vi "HFRR ADV v040.vi"() -> ()   [LabVIEW 2025] (continued)
            n2198 = Delete From Array(array=w2502, index=0) -> (array with subset deleted=w2408:dbl[])  [unwired: 1 in, 1 out]
            n2199 = Delete From Array(array=w2448, index=0) -> (array with subset deleted=w2404:dbl[])  [unwired: 1 in, 1 out]
            n2200 = Delete From Array(array=w2484, index=0) -> (array with subset deleted=w2406:dbl[])  [unwired: 1 in, 1 out]
            n2201 = Delete From Array(array=w2444, index=0) -> (array with subset deleted=w2402:dbl[])  [unwired: 1 in, 1 out]
            n2202 = Delete From Array(array=w2493, index=0) -> (array with subset deleted=w2407:dbl[])  [unwired: 1 in, 1 out]
            n2203 = Delete From Array(array=w2446, index=0) -> (array with subset deleted=w2403:dbl[])  [unwired: 1 in, 1 out]
            n2204 = Delete From Array(array=w2427, index=0) -> (array with subset deleted=w2399:dbl[])  [unwired: 1 in, 1 out]
            n2205 = Delete From Array(array=w2471, index=0) -> (array with subset deleted=w2457:dbl[])  [unwired: 1 in, 1 out]
            n2206 = Delete From Array(array=w2498, index=0) -> (array with subset deleted=w2459:dbl[])  [unwired: 1 in, 1 out]
            n2207 = Delete From Array(array=w2475, index=0) -> (array with subset deleted=w2405:dbl[])  [unwired: 1 in, 1 out]
            n2208 = Delete From Array(array=w2442, index=0) -> (array with subset deleted=w2401:dbl[])  [unwired: 1 in, 1 out]
            n2209 = Delete From Array(array=w2423, index=0) -> (array with subset deleted=w2397:dbl[])  [unwired: 1 in, 1 out]
            n2210 = Delete From Array(array=w2467, index=0) -> (array with subset deleted=w2455:dbl[])  [unwired: 1 in, 1 out]
            n2211 = Delete From Array(array=w2480, index=0) -> (array with subset deleted=w2460:dbl[])  [unwired: 1 in, 1 out]
            n2212 = Delete From Array(array=w2490, index=0) -> (array with subset deleted=w2373:dbl[])  [unwired: 1 in, 1 out]
            n2213 = Delete From Array(array=w2500, index=0) -> (array with subset deleted=w2375:dbl[])  [unwired: 1 in, 1 out]
            n2214 = Delete From Array(array=w2482, index=0) -> (array with subset deleted=w2371:dbl[])  [unwired: 1 in, 1 out]
            n2215 = Bundle "Bundle"(w2377, w2408) -> (w2395:cluster{dbl[], dbl[]})  [unwired: 1 in]
            n2216 = Bundle "Bundle"(w2377, w2462) -> (w2396:cluster{dbl[], dbl[]})  [unwired: 1 in]
            n2217 = Bundle "Bundle"(w2408, w2404) -> (w2410:cluster{dbl[], dbl[]})  [unwired: 1 in]
            n2218 = Bundle "Bundle"(w2373, w2372) -> (w2380:cluster{dbl[], dbl[]})  [unwired: 1 in]
            n2219 = Bundle "Bundle"(w2406, w2402) -> (w2412:cluster{dbl[], dbl[]})  [unwired: 1 in]
            n2220 = Bundle "Bundle"(w2373, w2406) -> (w2516:cluster{dbl[], dbl[]})  [unwired: 1 in]
            n2221 = Bundle "Bundle"(w2373, w2402) -> (w2440:cluster{dbl[], dbl[]})  [unwired: 1 in]
            n2222 = Bundle "Bundle"(w2373, w2461) -> (w2526:cluster{dbl[], dbl[]})  [unwired: 1 in]
            n2223 = Bundle "Bundle"(w2373, w2456) -> (w2464:cluster{dbl[], dbl[]})  [unwired: 1 in]
            n2224 = Bundle "Bundle"(w2373, w2487) -> (w2511:cluster{dbl[], dbl[]})  [unwired: 1 in]
            n2225 = Bundle "Bundle"(w2407, w2403) -> (w2411:cluster{dbl[], dbl[]})  [unwired: 1 in]
            n2226 = Bundle "Bundle"(w2375, w2374) -> (w2381:cluster{dbl[], dbl[]})  [unwired: 1 in]
            n2227 = Bundle "Bundle"(w2375, w2407) -> (w2518:cluster{dbl[], dbl[]})  [unwired: 1 in]
            n2228 = Bundle "Bundle"(w2375, w2403) -> (w2441:cluster{dbl[], dbl[]})  [unwired: 1 in]
            n2229 = Bundle "Bundle"(w2375, w2457) -> (w2465:cluster{dbl[], dbl[]})  [unwired: 1 in]
            n2230 = Bundle "Bundle"(w2375, w2459) -> (w2527:cluster{dbl[], dbl[]})  [unwired: 1 in]
            n2231 = Bundle "Bundle"(w2375, w2496) -> (w2509:cluster{dbl[], dbl[]})  [unwired: 1 in]
            n2232 = Bundle "Bundle"(w2405, w2401) -> (w2413:cluster{dbl[], dbl[]})  [unwired: 1 in]
            n2233 = Bundle "Bundle"(w2371, w2370) -> (w2379:cluster{dbl[], dbl[]})  [unwired: 1 in]
            n2234 = Bundle "Bundle"(w2371, w2405) -> (w2517:cluster{dbl[], dbl[]})  [unwired: 1 in]
            n2235 = Bundle "Bundle"(w2371, w2401) -> (w2439:cluster{dbl[], dbl[]})  [unwired: 1 in]
            n2236 = Bundle "Bundle"(w2371, w2455) -> (w2463:cluster{dbl[], dbl[]})  [unwired: 1 in]
            n2237 = Bundle "Bundle"(w2371, w2460) -> (w2525:cluster{dbl[], dbl[]})  [unwired: 1 in]
            n2238 = Bundle "Bundle"(w2371, w2478) -> (w2510:cluster{dbl[], dbl[]})  [unwired: 1 in]
            n2239 = call-poly <vilib>:"Mean.vi"("X"=w2458) -> ("mean"=→"CP1":dbl)  [unwired: 1 out]
            n2240 = call-poly <vilib>:"Mean.vi"("X"=w2399) -> ("mean"=→"КОФ2 3":dbl)  [unwired: 1 out]
            n2241 = call-poly <vilib>:"Mean.vi"("X"=w2457) -> ("mean"=→"CP2":dbl)  [unwired: 1 out]
            n2242 = call-poly <vilib>:"Mean.vi"("X"=w2459) -> ("mean"=→"КОФ2":dbl)  [unwired: 1 out]
            n2243 = call-poly <vilib>:"Mean.vi"("X"=w2397) -> ("mean"=→"КОФ2 5":dbl)  [unwired: 1 out]
            n2244 = call-poly <vilib>:"Mean.vi"("X"=w2455) -> ("mean"=→"CP4":dbl)  [unwired: 1 out]
            n2245 = call-poly <vilib>:"Mean.vi"("X"=w2460) -> ("mean"=→"КОФ4":dbl)  [unwired: 1 out]
            n2246 = Bundle "Bundle"(w2377, w2404) -> (w2368:cluster{dbl[], dbl[]})  [unwired: 1 in]
            n2247 = Bundle "Bundle"(w2377, w2458) -> (w2391:cluster{dbl[], dbl[]})  [unwired: 1 in]
            n2248 = Build Array "Build Array"(w2368, w2391) -> (w2394:cluster{dbl[], dbl[]}[])
            "XY Graph 17" <- w2394
            n2249 = Build Array "Build Array"(w2382, w2381, w2380, w2379) -> (→"Frequency ( Hz )":cluster{dbl[], dbl[]}[])
            n2250 = Build Array "Build Array"(w2410, w2411, w2412, w2413) -> (→"Air Temp ( °C ) vs Humidity ( % RH )":cluster{dbl[], dbl[]}[])
            n2251 = Build Array "Build Array"(w2395, w2518, w2516, w2517) -> (→"Air Temperature  ( °C )":cluster{dbl[], dbl[]}[])
            n2252 = Build Array "Build Array"(w2368, w2441, w2440, w2439) -> (→"Humidity ( %RH )":cluster{dbl[], dbl[]}[])
            n2253 = Build Array "Build Array"(w2396, w2527, w2526, w2525) -> (→"Coefficient Of Friction":cluster{dbl[], dbl[]}[])
            n2254 = Build Array "Build Array"(w2391, w2465, w2464, w2463) -> (→"Sample Temperature ( °C )":cluster{dbl[], dbl[]}[])
            n2255 = Build Array "Build Array"(w2369, w2509, w2511, w2510) -> (→"XY Graph 13":cluster{dbl[], dbl[]}[])
            n2256 = Bundle "Bundle"(w2377, w2400) -> (w2422:cluster{dbl[], dbl[]})  [unwired: 1 in]
            n2257 = Bundle "Bundle"(w2373, w2398) -> (w2420:cluster{dbl[], dbl[]})  [unwired: 1 in]
            n2258 = Bundle "Bundle"(w2375, w2399) -> (w2421:cluster{dbl[], dbl[]})  [unwired: 1 in]
            n2259 = Bundle "Bundle"(w2371, w2397) -> (w2419:cluster{dbl[], dbl[]})  [unwired: 1 in]
            n2260 = Build Array "Build Array"(w2422, w2421, w2420, w2419) -> (→"Stroke ( mm )":cluster{dbl[], dbl[]}[])
            n2261 = local write "XY Graph 16"(w2394) -> ()
          }
          frame #2 {
          }
          frame #3 {
            n2262 = local write "Numeric 8"(0 ("Numeric 8")) -> ()
            n2263 = local write "Numeric 11"(0 ("Numeric 11")) -> ()
            n2264 = local write "Numeric 12"(0 ("Numeric 12")) -> ()
            n2265 = local write "Numeric 13"(0 ("Numeric 13")) -> ()
            n2266 = property on="OPEN" class="Bool (strict)"("Visible"=TRUE) -> ()  [unwired: 2 in, 2 out]
            n2267 = local read "String Control 2"() -> (w2694:string)
            n2268 = local read "String Control 4"() -> (w2693:string)
            n2269 = local read "String Control 6"() -> (w2692:string)
            n2270 = local read "String Control 8"() -> (w2691:string)
            n2271 = Match Pattern(string=w2694, regular expression="Samples / cycle :- ") -> (after substring=w2708:string)  [unwired: 1 in, 3 out]
            n2272 = Match Pattern(string=w2694, regular expression="Frequency :- ") -> (after substring=w2727:string)  [unwired: 1 in, 3 out]
            n2273 = Match Pattern(string=w2693, regular expression="Samples / cycle :- ") -> (after substring=w2704:string)  [unwired: 1 in, 3 out]
            n2274 = Match Pattern(string=w2693, regular expression="Frequency :- ") -> (after substring=w2722:string)  [unwired: 1 in, 3 out]
            n2275 = Match Pattern(string=w2692, regular expression="Samples / cycle :- ") -> (after substring=w2700:string)  [unwired: 1 in, 3 out]
            n2276 = Match Pattern(string=w2692, regular expression="Frequency :- ") -> (after substring=w2717:string)  [unwired: 1 in, 3 out]
            n2277 = Match Pattern(string=w2691, regular expression="Samples / cycle :- ") -> (after substring=w2696:string)  [unwired: 1 in, 3 out]
            n2278 = Match Pattern(string=w2691, regular expression="Frequency :- ") -> (after substring=w2712:string)  [unwired: 1 in, 3 out]
            n2279 = String Subset(string=w2708, length (rest)=6 ("length (rest)")) -> (substring=w2710:string)  [unwired: 1 in]
            n2280 = String Subset(string=w2727, length (rest)=9 ("length (rest)")) -> (substring=w2729:string)  [unwired: 1 in]
            n2281 = String Subset(string=w2704, length (rest)=6 ("length (rest)")) -> (substring=w2706:string)  [unwired: 1 in]
            n2282 = String Subset(string=w2722, length (rest)=9 ("length (rest)")) -> (substring=w2724:string)  [unwired: 1 in]
            n2283 = String Subset(string=w2700, length (rest)=6 ("length (rest)")) -> (substring=w2702:string)  [unwired: 1 in]
            n2284 = String Subset(string=w2717, length (rest)=9 ("length (rest)")) -> (substring=w2719:string)  [unwired: 1 in]
            n2285 = String Subset(string=w2696, length (rest)=6 ("length (rest)")) -> (substring=w2698:string)  [unwired: 1 in]
            n2286 = String Subset(string=w2712, length (rest)=9 ("length (rest)")) -> (substring=w2714:string)  [unwired: 1 in]
            n2287 = Fract/Exp String To Number(string=w2710) -> (number=w2690:dbl)  [unwired: 3 in, 1 out]
            n2288 = Fract/Exp String To Number(string=w2729) -> (number=w2730:dbl)  [unwired: 3 in, 1 out]
            n2289 = Fract/Exp String To Number(string=w2706) -> (number=w2689:dbl)  [unwired: 3 in, 1 out]
            n2290 = Fract/Exp String To Number(string=w2724) -> (number=w2725:dbl)  [unwired: 3 in, 1 out]
            n2291 = Fract/Exp String To Number(string=w2702) -> (number=w2688:dbl)  [unwired: 3 in, 1 out]
            n2292 = Fract/Exp String To Number(string=w2719) -> (number=w2720:dbl)  [unwired: 3 in, 1 out]
            n2293 = Fract/Exp String To Number(string=w2698) -> (number=w2687:dbl)  [unwired: 3 in, 1 out]
            n2294 = Fract/Exp String To Number(string=w2714) -> (number=w2715:dbl)  [unwired: 3 in, 1 out]
            n2295 = local write "sample1"(w2690) -> ()
            n2296 = local write "freq1"(w2730) -> ()
            n2297 = local write "sample2"(w2689) -> ()
            n2298 = local write "freq2"(w2725) -> ()
            n2299 = local write "sample3"(w2688) -> ()
            n2300 = local write "freq3"(w2720) -> ()
            n2301 = local write "sample4"(w2687) -> ()
            n2302 = local write "freq 4"(w2715) -> ()
          }
        }
      }
    }
    n2303 = case shown="True" w2288 {
      selector: w2288 -> [_ w2307]
      frame False {
      }
      frame True {
        n2304 = Not(x=w2307) -> (.not. x?=w2303:bool)
        n2305 = local write "service 3"(w2303) -> ()
        n2306 = local write "OPEN 6"(w2303) -> ()
        n2307 = call <vilib>:"System Exec.vi"("wait until completion? (T)"=TRUE, "command line"="C:\\LAB-IQ\\Scar View.exe") -> ("error out"=→"error out 5":errorcluster)  [unwired: 6 in, 3 out]
      }
    }
    n2308 = case shown="\"Acquire\", Default" w2297 {
      frame "Acquire", Default {
        # "Elapsed time\ncof\nstroke\nAir temp\nTemp\nHumidity"
        n2309 = disable-structure shown="Disabled" {
          frame Disabled {
            n2310 = local read "Flag"() -> (w3006:dbl)
            n2311 = local read "RUN"() -> (w3003:bool)
            n2312 = Not(x=w3003) -> (.not. x?=w3002:bool)
            n2313 = Equal?(x=w3006, y=10.0) -> (x = y?=w3004:bool)
            n2314 = And(x=w3004, y=w3002) -> (x .and. y?=w3001:bool)
            n2315 = case shown="True" w3001 {
              frame False {
              }
              frame True {
                w3007 = FALSE ("Heater Button")
                n2316 = local write "Humidity"(w3007) -> ()
                n2317 = local write "Heater Button"(w3007) -> ()
              }
            }
          }
          frame Enabled {
          }
        }
        n2318 = disable-structure shown="Disabled" {
          frame Disabled {
            n2319 = case shown="True" {
              selector: _ -> [_ _]
              frame False {
              }
              frame True {
                w3052 = TRUE ("Heater")
                n2320 = local write "Humidity"(w3052) -> ()
                n2321 = local write "Heater Button"(w3052) -> ()
                n2322 = local read "TEST STANDARD"() -> (w3055:T3)
                n2323 = local read "TEST STANDARD"() -> (w3050:T3)
                n2324 = Equal?(x=w3055, y=enum16{"ASTM D6079", "ISO 12156", "Custom"}."ISO 12156" ("Test Standard")) -> (x = y?=w3053:bool)
                n2325 = Equal?(x=w3050, y=enum16{"ASTM D6079", "ISO 12156", "Custom"}."ASTM D6079" ("Test Standard")) -> (x = y?=w3049:bool)
                n2326 = case shown="True" w3053 {
                  frame False {
                  }
                  frame True {
                    n2327 = local write "airtempflg"(FALSE ("airtempflg")) -> ()
                    n2328 = local write item#-1(TRUE ("Heater")) -> ()
                  }
                }
                n2329 = case shown="True" w3049 {
                  frame False {
                  }
                  frame True {
                    n2330 = local write "airtempflg"(TRUE ("airtempflg")) -> ()
                    n2331 = local write item#-1(FALSE ("Heater")) -> ()
                  }
                }
              }
            }
          }
          frame Enabled {
          }
        }
        n2332 = stacked-sequence {
          frame #0 {
            n2333 = case shown="True" "RST FF" {
              frame False {
              }
              frame True {
                w3069 = 0.0 ("X Scale.Range:Maximum")
                n2334 = property on="Frictional Force ( N )" class="WFChart (strict)"("XScale.Maximum"=600.0 ("X Scale.Range:Maximum"), "XScale.Minimum"=w3069, "YScale.Maximum"=10.0 ("Y Scale.Range:Maximum"), "YScale.Minimum"=w3069) -> ()  [unwired: 2 in, 2 out]
              }
            }
          }
          frame #1 {
            n2335 = case shown="True" "RST TEMP" {
              frame False {
              }
              frame True {
                n2336 = property on="Temperature ( Deg C )" class="WFChart (strict)"("XScale.Minimum"=0.0 ("X Scale.Range:Minimum"), "XScale.Maximum"=600.0 ("X Scale.Range:Maximum"), "YScale.Minimum"=0.0 ("Y Scale.Range:Minimum"), "YScale.Maximum"=100.0 ("Y Scale.Range:Maximum")) -> ()  [unwired: 2 in, 2 out]
              }
            }
          }
          frame #2 {
            n2337 = case shown="True" "RSTCOF" {
              frame False {
              }
              frame True {
                n2338 = property on="Coefficient of Friction" class="WFChart (strict)"("XScale.Minimum"=0.0 ("X Scale.Range:Minimum"), "XScale.Maximum"=600.0 ("X Scale.Range:Maximum"), "YScale.Maximum"=1.0 ("X Scale.Range:Minimum"), "YScale.Minimum"=0.0 ("X Scale.Range:Minimum")) -> ()  [unwired: 2 in, 2 out]
              }
            }
          }
          frame #3 {
            n2339 = case shown="True" "RSTCOF 2" {
              frame False {
              }
              frame True {
                (unwired) 100.0 ("Y Scale.Range:Maximum")
                (unwired) 0.0 ("Y Scale.Range:Minimum")
                (unwired) 600.0 ("X Scale.Range:Maximum")
                (unwired) 0.0 ("X Scale.Range:Minimum")
              }
            }
          }
          frame #4 {
            n2340 = case shown="True" "RSTCOF 3" {
              frame False {
              }
              frame True {
                n2341 = property on="Electrical Contact Resistance ( % )" class="WFChart (strict)"("XScale.Minimum"=0.0 ("X Scale.Range:Minimum"), "XScale.Maximum"=600.0 ("X Scale.Range:Maximum"), "YScale.Minimum"=0.0 ("Y Scale.Range:Minimum"), "YScale.Maximum"=100.0 ("Y Scale.Range:Maximum")) -> ()  [unwired: 2 in, 2 out]
              }
            }
          }
        }
        n2342 = local read "RUN"() -> (w2996:bool)
        n2343 = case shown="False" w2996 {
          frame False {
          }
          frame True {
          }
        }
        n2344 = local read "RUN"() -> (w3000:bool)
        n2345 = case shown="False" w3000 {
          tunnel: [FALSE ("TEST RUNNING") TRUE ("TEST RUNNING")] -> w2999
          frame False {
            w3088 = 0.0 ("Flag")
            n2346 = local write "Elapsed time"(0.0 ("elapsedtime")) -> ()
            n2347 = local write "Time Remaining"(w3088) -> ()
            n2348 = local write "Flag"(w3088) -> ()
            n2349 = local write "Remaining Time"(w3088) -> ()
          }
          frame True {
            n2350 = local write "Flag"(10.0 ("Flag")) -> ()
          }
        }
        n2351 = local read "AIR TEMP"() -> (w2994:dbl)
        n2352 = Greater Or Equal?(x=w2994, y=15.0) -> (x >= y?=w2995:bool)
        "powstat" <- w2995
        n2353 = case shown="True" "Save & Continue" {
          frame False {
          }
          frame True {
            n2354 = local read "USER ID"() -> (w3392:string)
            n2355 = local read "FILE"() -> (w3400:string)
            n2356 = String Length(string=w3400) -> (length=w3398:i32)
            n2357 = String Length(string=w3392) -> (length=w3395:i32)
            n2358 = Greater?(x=w3398, y=0) -> (0:w3397:bool)
            n2359 = Greater?(x=w3395, y=0) -> (0:w3394:bool)
            n2360 = And(x=w3397, y=w3394) -> (x .and. y?=w3393:bool)
            n2361 = case shown="True" w3393 {
              frame False {
                n2362 = stacked-sequence {
                  frame #0 {
                    n2363 = One Button Dialog(message="Please Enter a File Name and Operator ID to save data !", button name ("OK")="Ok") -> ()  [unwired: 1 out]
                  }
                  frame #1 {
                    n2364 = local write "Save & Continue"(FALSE ("OK Button")) -> ()
                  }
                }
                n2365 = local write "Save & Continue"(FALSE ("OK Button")) -> ()
              }
              frame True {
                n2366 = stacked-sequence {
                  frame #0 {
                    n2367 = local read "FILE"() -> (w3406:string)
                    n2368 = call "file check.vi"("file name in"=w3406) -> ("file name out"=w3405:string)  [unwired: 9 in, 1 out]
                    n2369 = call <vilib>:"Application Directory.vi"() -> ("Application Directory"=w3416:path)
                    n2370 = Build Path(base path=w3416, name or relative path="data") -> (appended path=w3415:path)
                    n2371 = call <vilib>:"Trim Whitespace.vi"("string"=w3405) -> ("trimmed string"=w3413:string)  [unwired: 1 in]
                    n2372 = call <vilib>:"Trim Whitespace.vi"("string"=w3405) -> ("trimmed string"=w3414:string)  [unwired: 1 in]
                    n2373 = List Folder(path=w3415) -> (folder names=w3411:string[])  [unwired: 3 in, 3 out]
                    n2374 = Match Pattern(string=w3413, regular expression="_(") -> (before substring=w3410:string)  [unwired: 1 in, 3 out]
                    n2375 = for {
                      tunnel: w3411 -> [w3425] mode=indexing
                      tunnel: w3410 -> [w3423]
                      shift-right: [w3421] -> w3408
                      shift-left: bool[] [] -> [w3422]
                      n2376 = Match Pattern(string=w3425, regular expression="_(") -> (before substring=w3424:string)  [unwired: 1 in, 3 out]
                      n2377 = Equal?(x=w3424, y=w3423) -> (x = y?=w3420:bool)
                      n2378 = case shown="True" w3420 {
                        tunnel: w3420 -> [_ w3428]
                        tunnel: w3422 -> [w3427 w3430]
                        tunnel: [w3427 w3429] -> w3421
                        frame False {
                        }
                        frame True {
                          n2379 = Insert Into Array(array=w3430, new element=w3428) -> (w3429:bool[])  [unwired: 1 in]
                        }
                      }
                    }
                    n2380 = Equal?(x=w3411, y=w3410) -> (x = y?=w3419:bool[])
                    n2381 = Or Array Elements(Boolean array=w3419) -> (logical OR=w3418:bool)
                    n2382 = Array Size(array=w3408) -> (size(s)=w3407:i32)
                    n2383 = case shown="True" w3418 {
                      tunnel: w3414 -> [_ w3438]
                      tunnel: w3407 -> [_ w3431]
                      frame False {
                      }
                      frame True {
                        n2384 = Number To Decimal String(number=w3431) -> (decimal integer string=w3434:string)  [unwired: 1 in]
                        n2385 = Search/Split String(string=w3438, search string/char (-)="_(" ("regular expression")) -> (substring before match=w3436:string)  [unwired: 1 in, 2 out]
                        n2386 = Concatenate Strings(w3436, "_(" ("regular expression"), w3434, ")" ("regular expression")) -> (w3432:string)
                        n2387 = local write "FILE"(w3432) -> ()
                      }
                    }
                  }
                  frame #1 {
                    w3441 = 0.0
                    w3454 = cluster{"y":dbl, dbl, "y":dbl}[] [] ("History Data")
                    w3455 = FALSE ("Heater Button")
                    (unwired) ")!" ("string")
                    (unwired) ")" ("string")
                    w3453 = dbl[] [] ("History Data")
                    w3459 = "\r"
                    # "C:\\WinDucom\\Data\\"
                    # "C:\\LAB-IQ-NXT\\data"
                    n2388 = local write "Humidity ( %RH )"(w3441) -> ()
                    n2389 = local write "Frequency ( Hz )"(w3441) -> ()
                    n2390 = local write "Stroke 3"(w3441) -> ()
                    n2391 = local write "speedop"(0.0 ("PIDclk 2")) -> ()
                    n2392 = local write "Set Temp 2"(65.0 ("Set Temp 2")) -> ()
                    n2393 = local write "AIR TEMP"(w3441) -> ()
                    n2394 = local write "clk"(0.0 ("clk")) -> ()
                    n2395 = local write "Stroke 4"(w3441) -> ()
                    n2396 = local write "COF 2"(w3441) -> ()
                    n2397 = local write "TEMP"(w3441) -> ()
                    n2398 = local write "ecr 3"(w3441) -> ()
                    n2399 = local write "FF 3"(w3441) -> ()
                    n2400 = local write "FF 2"(w3441) -> ()
                    n2401 = property on="Coefficient of Friction" class="WFChart (strict)"("History Data"=w3453) -> ()  [unwired: 2 in, 2 out]
                    n2402 = property on="Coefficient of Friction" class="WFChart (strict)"("History Data"=w3453) -> ()  [unwired: 2 in, 2 out]
                    n2403 = property on="Frictional Force ( N )" class="WFChart (strict)"("History Data"=w3453) -> ()  [unwired: 2 in, 2 out]
                    n2404 = property on="Electrical Contact Resistance ( % )" class="WFChart (strict)"("History Data"=w3453) -> ()  [unwired: 2 in, 2 out]
                    n2405 = property on="Electrical Contact Resistance ( % )" class="WFChart (strict)"("History Data"=w3453) -> ()  [unwired: 2 in, 2 out]
                    n2406 = property on="Temperature ( Deg C )" class="WFChart (strict)"("History Data"=w3453) -> ()  [unwired: 2 in, 2 out]
                    n2407 = property on="Frictional Force ( N )" class="WFChart (strict)"("History Data"=w3453) -> ()  [unwired: 2 in, 2 out]
                    n2408 = property on="Coefficient of Friction" class="WFChart (strict)"("History Data"=w3453) -> ()  [unwired: 2 in, 2 out]
                    n2409 = property on="Frictional Force ( N )" class="WFChart (strict)"("History Data"=w3453) -> ()  [unwired: 2 in, 2 out]
                    n2410 = property on="Electrical Contact Resistance ( % )" class="WFChart (strict)"("History Data"=w3453) -> ()  [unwired: 2 in, 2 out]
                    n2411 = property on="Temperature ( Deg C )" class="WFChart (strict)"("History Data"=w3453) -> ()  [unwired: 2 in, 2 out]
                    n2412 = property on="Stroke ( mm )" class="WFChart (strict)"("History Data"=w3454) -> ()  [unwired: 2 in, 2 out]
                    n2413 = property on="Stroke ( mm )" class="WFChart (strict)"("History Data"=w3454) -> ()  [unwired: 2 in, 2 out]
                    n2414 = local write "Humidity"(w3455) -> ()
                    n2415 = local write "Heater Button"(w3455) -> ()
                    n2416 = local read "FILE"() -> (w3449:string)
                    n2417 = disable-structure shown="Enabled" {
                      disable-tunnel: [w3493 _] -> w3440
                      frame Enabled {
                        n2418 = local read "NORMAL LOAD"() -> (w3493:dbl)
                      }
                      frame Disabled {
                      }
                    }
                    n2419 = call "file check.vi"("file name in"=w3449) -> ("error out"=w3452:errorcluster, "file name out"=w3446:string)  [unwired: 9 in]
                    n2420 = call "FILE PATH CREATION.vi"("error in"=w3452, "FILE NAME :"=w3446) -> ("FILE OUT"=w3445:path)  [unwired: 8 in, 1 out]
                    n2421 = Concatenate Strings(w3446, ".dgf" ("Substring")) -> (w3451:string)
                    n2422 = Concatenate Strings(w3446, ".duf" ("Substring")) -> (w3447:string)
                    n2423 = Multiply(x=w3440, y=1.0) -> (x*y=w3472:dbl)
                    n2424 = Build Path(base path=w3445, name or relative path=w3451) -> (appended path=w3444:path)
                    n2425 = Build Path(base path=w3445, name or relative path=w3447) -> (appended path=w3443:path)
                    n2426 = Number To Fractional String(number=w3472, width (-)=i16 5, precision (6)=i16 2) -> (F-format string=w3480:string)  [unwired: 1 in]
                    n2427 = local read "tested by"() -> (w3439:string)
                    n2428 = local read "Fuel Discription :"() -> (w3468:string)
                    n2429 = local read "Batch Ref Num :"() -> (w3457:string)
                    n2430 = Get Date/Time String(date format (0)=enum16{"short", "long", "abbreviated"}."short") -> (date string=w3491:string, time string=w3488:string)  [unwired: 2 in]
                    n2431 = local read "Remarks :"() -> (w3467:string)
                    n2432 = Concatenate Strings("Load :- " ("Substring"), w3480, " grams ," ("Substring")) -> (w3479:string)
                    n2433 = local read "String 41"() -> (w3460:string)
                    n2434 = Concatenate Strings(w3468) -> (w3469:string)
                    n2435 = Concatenate Strings(w3457) -> (w3456:string)
                    n2436 = Concatenate Strings(w3439) -> (w3463:string)
                    n2437 = Concatenate Strings("(" ("Substring"), w3491, ")" ("Substring"), w3488) -> (w3462:string)
                    "concatenated string" <- w3462
                    n2438 = Concatenate Strings(w3467, "," ("string")) -> (w3466:string)
                    n2439 = Concatenate Strings("  TIME;      COF;       STROKE;     AIR TEMP;  TEMP;  HUMIDITY;  ECR; PID-OUT; FREQUENCY" ("Substring"), "\r") -> (w3475:string)
                    n2440 = Concatenate Strings(w3460, w3459, "Fuel Discription :-" ("Substring"), w3469, w3459, w3479, w3459, "Batch Ref Num :-" ("Substring"), w3456, w3459, " Remarks :- " ("Substring"), w3466, w3459, " Date :- " ("Substring"), w3462, w3459, "Tested By :-" ("Substring"), w3463) -> (w3473:string)
                    "REMARKS" <- w3473
                    n2441 = call <vilib>:"Write Characters To File.vi"("append to file? (new file:F)"=FALSE, "character string"=w3475, "file path (dialog if empty)"=w3444) -> ()  [unwired: 2 in, 1 out]
                    n2442 = call <vilib>:"Write Characters To File.vi"("append to file? (new file:F)"=FALSE, "character string"=w3473, "file path (dialog if empty)"=w3443) -> ()  [unwired: 2 in, 1 out]
                  }
                  frame #2 {
                    n2443 = local write "Cycles elapsed"(0 ("Cycles elapsed")) -> ()
                    n2444 = local write "cyclecount"(0 ("cyclecount")) -> ()
                    n2445 = local write "Save & Continue"(FALSE ("OK")) -> ()
                    n2446 = local write "autostrtflg"(TRUE ("autostrtflg")) -> ()
                    n2447 = local write "Save"(FALSE ("Save")) -> ()
                    n2448 = Get Date/Time In Seconds() -> (seconds since 1Jan1904=w3498:timestamp)
                    n2449 = To Double Precision Float(number=w3498) -> (double precision float=w3497:dbl)
                    n2450 = local write "acq timer"(w3497) -> ()
                    n2451 = One Button Dialog(message="Please ensure sample is mounted properly and machine is ready in all aspects for testing !", button name ("OK")="Ok") -> ()  [unwired: 1 out]
                  }
                  frame #3 {
                    n2452 = stacked-sequence {
                      frame #0 {
                        n2453 = local write "Main Dashboard Buttons"(T1."Dashboard" ("Main Dashboard Buttons")) -> ()
                        n2454 = local write "Main Tab"(T2."Acquire" ("Main Tab")) -> ()
                      }
                      frame #1 {
                        n2455 = local write "EVENT LOG"("" ("EVENT LOG")) -> ()
                      }
                      frame #2 {
                        n2456 = Wait (ms)(milliseconds to wait=u32 50) -> ()  [unwired: 1 out]
                      }
                      frame #3 {
                        n2457 = disable-structure shown="Disabled" {
                          frame Disabled {
                            n2458 = local read "EVENT LOG"() -> (w3510:string)
                            n2459 = call "Event Log.vi"("Content"="Test Details", "EVENT LOG"=w3510) -> ("EVENT LOG"=w3509:string)  [unwired: 8 in, 1 out]
                            n2460 = local write "EVENT LOG"(w3509) -> ()
                          }
                          frame Enabled {
                          }
                        }
                      }
                      frame #4 {
                        n2461 = Wait (ms)(milliseconds to wait=u32 50) -> ()  [unwired: 1 out]
                      }
                      frame #5 {
                        n2462 = local read "FILE"() -> (w3512:string)
                        n2463 = Concatenate Strings("File Name :" ("Content"), w3512) -> (w3513:string)
                        n2464 = local read "EVENT LOG"() -> (w3516:string)
                        n2465 = call "Event Log.vi"("Content"=w3513, "EVENT LOG"=w3516) -> ("EVENT LOG"=w3515:string)  [unwired: 8 in, 1 out]
                        n2466 = local write "EVENT LOG"(w3515) -> ()
                      }
                      frame #6 {
                        n2467 = Wait (ms)(milliseconds to wait=u32 50) -> ()  [unwired: 1 out]
                      }
                      frame #7 {
                        n2468 = local read "Batch Ref Num :"() -> (w3518:string)
                        n2469 = Concatenate Strings("Batch Ref No :" ("Content"), w3518) -> (w3519:string)
                        n2470 = local read "EVENT LOG"() -> (w3522:string)
                        n2471 = call "Event Log.vi"("Content"=w3519, "EVENT LOG"=w3522) -> ("EVENT LOG"=w3521:string)  [unwired: 8 in, 1 out]
                        n2472 = local write "EVENT LOG"(w3521) -> ()
                      }
                      frame #8 {
                        n2473 = Wait (ms)(milliseconds to wait=u32 50) -> ()  [unwired: 1 out]
                      }
                      frame #9 {
                        n2474 = local read "tested by"() -> (w3524:string)
                        n2475 = Concatenate Strings("Tested By :" ("Content"), w3524) -> (w3525:string)
                        n2476 = local read "EVENT LOG"() -> (w3528:string)
                        n2477 = call "Event Log.vi"("Content"=w3525, "EVENT LOG"=w3528) -> ("EVENT LOG"=w3527:string)  [unwired: 8 in, 1 out]
                        n2478 = local write "EVENT LOG"(w3527) -> ()
                      }
                      frame #10 {
                        n2479 = Wait (ms)(milliseconds to wait=u32 50) -> ()  [unwired: 1 out]
                      }
                      frame #11 {
                        n2480 = local read "TEST STANDARD"() -> (w3531:T3)
                        n2481 = case shown="\"ASTM D6079\", Default" w3531 {
                          tunnel: ["ASTM D6079" "ISO 12156" "CEC F-096-A-06" "Custom"] -> w3530
                          frame "ASTM D6079", Default {
                          }
                          frame "ISO 12156" {
                          }
                          frame "CEC F-096-A-06" {
                          }
                          frame "Custom" {
                          }
                        }
                        n2482 = Concatenate Strings("Test Standard :" ("Content"), w3530) -> (w3532:string)
                        n2483 = local read "EVENT LOG"() -> (w3535:string)
                        n2484 = call "Event Log.vi"("Content"=w3532, "EVENT LOG"=w3535) -> ("EVENT LOG"=w3534:string)  [unwired: 8 in, 1 out]
                        n2485 = local write "EVENT LOG"(w3534) -> ()
                      }
                      frame #12 {
                        n2486 = Wait (ms)(milliseconds to wait=u32 50) -> ()  [unwired: 1 out]
                      }
                      frame #13 {
                        n2487 = local read "Fuel Discription :"() -> (w3541:string)
                        n2488 = Concatenate Strings("Fuel Description :" ("Content"), w3541) -> (w3542:string)
                        n2489 = local read "EVENT LOG"() -> (w3545:string)
                        n2490 = call "Event Log.vi"("Content"=w3542, "EVENT LOG"=w3545) -> ("EVENT LOG"=w3544:string)  [unwired: 8 in, 1 out]
                        n2491 = local write "EVENT LOG"(w3544) -> ()
                      }
                      frame #14 {
                        n2492 = Wait (ms)(milliseconds to wait=u32 50) -> ()  [unwired: 1 out]
                      }
                      frame #15 {
                        n2493 = local read "Remarks :"() -> (w3547:string)
                        n2494 = Concatenate Strings("Remarks :" ("Content"), w3547) -> (w3548:string)
                        n2495 = local read "EVENT LOG"() -> (w3551:string)
                        n2496 = call "Event Log.vi"("Content"=w3548, "EVENT LOG"=w3551) -> ("EVENT LOG"=w3550:string)  [unwired: 8 in, 1 out]
                        n2497 = local write "EVENT LOG"(w3550) -> ()
                      }
                      frame #16 {
                        n2498 = Wait (ms)(milliseconds to wait=u32 50) -> ()  [unwired: 1 out]
                      }
                      frame #17 {
                        n2499 = local read "USER ID"() -> (w3553:string)
                        n2500 = Concatenate Strings("Operator ID :" ("Content"), w3553) -> (w3555:string)
                        n2501 = local read "EVENT LOG"() -> (w3557:string)
                        n2502 = call "Event Log.vi"("Content"=w3555, "EVENT LOG"=w3557) -> ("EVENT LOG"=w3556:string)  [unwired: 8 in, 1 out]
                        n2503 = local write "EVENT LOG"(w3556) -> ()
                      }
                      frame #18 {
                        n2504 = Wait (ms)(milliseconds to wait=u32 50) -> ()  [unwired: 1 out]
                      }
                      frame #19 {
                        n2505 = disable-structure shown="Disabled" {
                          frame Disabled {
                            n2506 = local read "EVENT LOG"() -> (w3561:string)
                            n2507 = call "Event Log.vi"("Content"="Test Parameter", "EVENT LOG"=w3561) -> ("EVENT LOG"=w3560:string)  [unwired: 8 in, 1 out]
                            n2508 = local write "EVENT LOG"(w3560) -> ()
                          }
                          frame Enabled {
                          }
                        }
                      }
                      frame #20 {
                        n2509 = Wait (ms)(milliseconds to wait=u32 50) -> ()  [unwired: 1 out]
                      }
                      frame #21 {
                        n2510 = local read "Set Hz"() -> (w3565:dbl)
                        n2511 = Number To Fractional String(number=w3565, precision (6)=i16 2) -> (F-format string=w3564:string)  [unwired: 2 in]
                        n2512 = Concatenate Strings("Set Frequency [Hz] :" ("Content"), w3564) -> (w3567:string)
                        n2513 = local read "EVENT LOG"() -> (w3569:string)
                        n2514 = call "Event Log.vi"("Content"=w3567, "EVENT LOG"=w3569) -> ("EVENT LOG"=w3568:string)  [unwired: 8 in, 1 out]
                        n2515 = local write "EVENT LOG"(w3568) -> ()
                      }
                      frame #22 {
                        n2516 = Wait (ms)(milliseconds to wait=u32 50) -> ()  [unwired: 1 out]
                      }
                      frame #23 {
                        n2517 = local read "NORMAL LOAD"() -> (w3572:dbl)
                        n2518 = Number To Fractional String(number=w3572, precision (6)=i16 2) -> (F-format string=w3573:string)  [unwired: 2 in]
                        n2519 = Concatenate Strings("Applied Load [grams] :" ("Content"), w3573) -> (w3575:string)
                        n2520 = local read "EVENT LOG"() -> (w3577:string)
                        n2521 = call "Event Log.vi"("Content"=w3575, "EVENT LOG"=w3577) -> ("EVENT LOG"=w3576:string)  [unwired: 8 in, 1 out]
                        n2522 = local write "EVENT LOG"(w3576) -> ()
                      }
                      frame #24 {
                        n2523 = Wait (ms)(milliseconds to wait=u32 50) -> ()  [unwired: 1 out]
                      }
                      frame #25 {
                        n2524 = local read "Set Strk"() -> (w3580:dbl)
                        n2525 = Number To Fractional String(number=w3580, precision (6)=i16 2) -> (F-format string=w3581:string)  [unwired: 2 in]
                        n2526 = Concatenate Strings("Set Stroke [mm] :" ("Content"), w3581) -> (w3583:string)
                        n2527 = local read "EVENT LOG"() -> (w3585:string)
                        n2528 = call "Event Log.vi"("Content"=w3583, "EVENT LOG"=w3585) -> ("EVENT LOG"=w3584:string)  [unwired: 8 in, 1 out]
                        n2529 = local write "EVENT LOG"(w3584) -> ()
                      }
                      frame #26 {
                        n2530 = Wait (ms)(milliseconds to wait=u32 50) -> ()  [unwired: 1 out]
                      }
                      frame #27 {
                        n2531 = local read "Set Temp"() -> (w3588:dbl)
                        n2532 = Number To Fractional String(number=w3588, precision (6)=i16 2) -> (F-format string=w3589:string)  [unwired: 2 in]
                        n2533 = Concatenate Strings("Set Temperature [deg C] :" ("Content"), w3589) -> (w3591:string)
                        n2534 = local read "EVENT LOG"() -> (w3593:string)
                        n2535 = call "Event Log.vi"("Content"=w3591, "EVENT LOG"=w3593) -> ("EVENT LOG"=w3592:string)  [unwired: 8 in, 1 out]
                        n2536 = local write "EVENT LOG"(w3592) -> ()
                      }
                      frame #28 {
                        n2537 = Wait (ms)(milliseconds to wait=u32 50) -> ()  [unwired: 1 out]
                      }
                      frame #29 {
                        n2538 = local read "Set Rh"() -> (w3596:dbl)
                        n2539 = Number To Fractional String(number=w3596, precision (6)=i16 2) -> (F-format string=w3597:string)  [unwired: 2 in]
                        n2540 = Concatenate Strings("Set Humidity [%RH] :" ("Content"), w3597) -> (w3599:string)
                        n2541 = local read "EVENT LOG"() -> (w3601:string)
                        n2542 = call "Event Log.vi"("Content"=w3599, "EVENT LOG"=w3601) -> ("EVENT LOG"=w3600:string)  [unwired: 8 in, 1 out]
                        n2543 = local write "EVENT LOG"(w3600) -> ()
                      }
                      frame #30 {
                        n2544 = Wait (ms)(milliseconds to wait=u32 50) -> ()  [unwired: 1 out]
                      }
                      frame #31 {
                        n2545 = local read "test time"() -> (w3604:dbl)
                        n2546 = Number To Fractional String(number=w3604, precision (6)=i16 1) -> (F-format string=w3605:string)  [unwired: 2 in]
                        n2547 = Concatenate Strings("Test Duration [mins] :" ("Content"), w3605) -> (w3607:string)
                        n2548 = local read "EVENT LOG"() -> (w3609:string)
                        n2549 = call "Event Log.vi"("Content"=w3607, "EVENT LOG"=w3609) -> ("EVENT LOG"=w3608:string)  [unwired: 8 in, 1 out]
                        n2550 = local write "EVENT LOG"(w3608) -> ()
                      }
                      frame #32 {
                        w3610 = dbl[] [] ("History Data")
                        w3611 = cluster{"y":dbl, dbl, "y":dbl}[] [] ("History Data")
                        w3612 = FALSE ("Visible")
                        n2551 = property on="Stroke ( mm )" class="WFChart (strict)"("History Data"=w3611) -> ()  [unwired: 2 in, 2 out]
                        n2552 = property on="Temperature ( Deg C )" class="WFChart (strict)"("History Data"=w3610) -> ()  [unwired: 2 in, 2 out]
                        n2553 = property on="Electrical Contact Resistance ( % )" class="WFChart (strict)"("History Data"=w3610) -> ()  [unwired: 2 in, 2 out]
                        n2554 = property on="Coefficient of Friction" class="WFChart (strict)"("History Data"=w3610) -> ()  [unwired: 2 in, 2 out]
                        n2555 = property on="Frictional Force ( N )" class="WFChart (strict)"("History Data"=w3610) -> ()  [unwired: 2 in, 2 out]
                        n2556 = property on="Coefficient of Friction" class="WFChart (strict)"("History Data"=w3610) -> ()  [unwired: 2 in, 2 out]
                        n2557 = property on="Frictional Force ( N )" class="WFChart (strict)"("History Data"=w3610) -> ()  [unwired: 2 in, 2 out]
                        n2558 = property on="Electrical Contact Resistance ( % )" class="WFChart (strict)"("History Data"=w3610) -> ()  [unwired: 2 in, 2 out]
                        n2559 = property on="Stroke ( mm )" class="WFChart (strict)"("History Data"=w3611) -> ()  [unwired: 2 in, 2 out]
                        n2560 = property on="Temperature ( Deg C )" class="WFChart (strict)"("History Data"=w3610) -> ()  [unwired: 2 in, 2 out]
                        n2561 = property on="Service Password Log" class="Str"("Visible"=w3612) -> ()  [unwired: 2 in, 2 out]
                        n2562 = property on="Password 3" class="Clust (strict)"("Visible"=w3612) -> ()  [unwired: 2 in, 2 out]
                      }
                    }
                    "TEST FILE NAM,E SAVED" <- TRUE ("TEST FILE NAM,E SAVED")
                  }
                }
              }
            }
          }
        }
        n2563 = local write "Test \nStatus"(w2999) -> ()
        n2564 = local write "Save"(w2999) -> ()
        n2565 = local read "Main Tab"() -> (w2993:T2)
        n2566 = case shown="True" w2996 {
          frame False {
            n2567 = local read "Rt 3"() -> (w3060:bool)
            n2568 = case shown="True" w3060 {
              frame False {
              }
              frame True {
                n2569 = local write "Rt 3"(FALSE ("Rt 3")) -> ()
              }
            }
            "Rt" <- TRUE ("Rt")
            "Rt 2" <- FALSE ("Rt")
          }
          frame True {
            n2570 = local read "Rt"() -> (w3066:bool)
            n2571 = local write "Rt 2"(TRUE ("Rt 2")) -> ()
            n2572 = case shown="True" w3066 {
              frame False {
              }
              frame True {
                n2573 = local write "Rt"(FALSE ("Rt")) -> ()
              }
            }
            "Rt 3" <- TRUE ("Rt 3")
          }
        }
        n2574 = case shown="\"Acquire\"" w2993 {
          tunnel: w2995 -> [_ w3095]
          frame Default {
            w3094 = 0.0 ("output")
            n2575 = local write "PID-out"(w3094) -> ()
            n2576 = local write "Frequency ( Hz )"(w3094) -> ()
            n2577 = local write "STROKE Initialize"(TRUE ("STROKE Initialize")) -> ()
          }
          frame "Acquire" {
            n2578 = stacked-sequence {
              frame #0 {
                n2579 = local read "Auto Start Test"() -> (w3097:bool)
                n2580 = case shown="True" w3097 {
                  tunnel: "RUN" -> [w3118 w3121]
                  tunnel: [w3118 w3120] -> w3098
                  frame False {
                  }
                  frame True {
                    n2581 = local read "Auto Start Temp"() -> (w3119:bool)
                    n2582 = Or(x=w3121, y=w3119) -> (x .or. y?=w3120:bool)
                  }
                }
                n2583 = local read "clk"() -> (w3117:dbl)
                n2584 = local read "Save"() -> (w3113:bool)
                n2585 = Equal?(x=w3117, y=0.0) -> (x = y?=w3114:bool)
                n2586 = And(x=w3114, y=w3113) -> (x .and. y?=w3115:bool)
                n2587 = Not(x="Engage") -> (.not. x?=w3104:bool)
                n2588 = case shown="False" w3098 {
                  tunnel: [0.0 w3145] -> w3100
                  frame False {
                    (unwired) TRUE ("Visible")
                    n2589 = local read "Auto Start Test"() -> (w3125:bool)
                    n2590 = local write "Start Time"(TRUE ("Start Time")) -> ()
                    n2591 = property on="Stroke 2" class="DigNum (strict)"("Visible"=FALSE) -> ()  [unwired: 2 in, 2 out]
                    n2592 = case shown="False" w3125 {
                      frame False {
                        n2593 = property on="Heater Button" class="Bool (strict)"("DisabledEnum"=T19."Enabled" ("Disabled")) -> ()  [unwired: 2 in, 2 out]
                        n2594 = property on="Humidity" class="Bool (strict)"("DisabledEnum"=T19."Enabled" ("Disabled")) -> ()  [unwired: 2 in, 2 out]
                      }
                      frame True {
                      }
                    }
                    n2595 = case shown="False" "TestCompFlg" {
                      frame False {
                        n2596 = local read "StartFlg"() -> (w3133:bool)
                        n2597 = case shown="True" w3133 {
                          frame False {
                          }
                          frame True {
                            n2598 = stacked-sequence {
                              frame #0 {
                                n2599 = local read "EVENT LOG"() -> (w3137:string)
                                n2600 = call "Event Log.vi"("Content"="Test was interrupted", "EVENT LOG"=w3137) -> ("EVENT LOG"=w3138:string)  [unwired: 8 in, 1 out]
                                n2601 = local write "EVENT LOG"(w3138) -> ()
                                n2602 = property on="RUN" class="Bool (strict)"("Visible"=TRUE) -> ()  [unwired: 2 in, 2 out]
                                n2603 = property on="Auto Start Test" class="Bool (strict)"("Visible"=TRUE) -> ()  [unwired: 2 in, 2 out]
                              }
                              frame #1 {
                                w3141 = FALSE ("StartFlg")
                                n2604 = property on="Heater Button" class="Bool (strict)"("Val(Sgnl)"=FALSE ("Value (Signaling)")) -> ()  [unwired: 2 in, 2 out]
                                n2605 = local write "Heater Button"(w3141) -> ()
                                n2606 = local write "StartFlg"(w3141) -> ()
                                n2607 = local write "Humidity"(w3141) -> ()
                                n2608 = local write "Humidity 2"(TRUE ("Humidity")) -> ()
                              }
                              frame #2 {
                                n2609 = local write "Due Write"("VC;0" ("Command")) -> ()
                              }
                              frame #3 {
                                n2610 = Wait (ms)(milliseconds to wait=u32 1500) -> ()  [unwired: 1 out]
                              }
                              frame #4 {
                                n2611 = local write "Due Write"("HE;0" ("Command")) -> ()
                              }
                            }
                          }
                        }
                      }
                      frame True {
                      }
                    }
                    n2612 = local write "String 14"("Test will autostart once parameters reach the set value." ("String 14")) -> ()
                  }
                  frame True {
                    (unwired) FALSE ("Visible")
                    n2613 = property on="Stroke 2" class="DigNum (strict)"("Visible"=TRUE) -> ()  [unwired: 2 in, 2 out]
                    n2614 = property on="STOP 2" class="Bool (strict)"("Disabled"=u8 2) -> ()  [unwired: 2 in, 2 out]
                    n2615 = local write "String 14"(" Running....." ("String 14")) -> ()
                    n2616 = property on="Heater Button" class="Bool (strict)"("DisabledEnum"=T19."Disabled and Grayed Out" ("Disabled")) -> ()  [unwired: 2 in, 2 out]
                    n2617 = property on="Humidity" class="Bool (strict)"("DisabledEnum"=T19."Disabled and Grayed Out" ("Disabled")) -> ()  [unwired: 2 in, 2 out]
                    n2618 = case shown="True" "Start Time" {
                      selector: "Start Time" -> [_ w3164]
                      frame False {
                      }
                      frame True {
                        n2619 = Not(x=w3164) -> (.not. x?=w3163:bool)
                        n2620 = local write "Start Time"(w3163) -> ()
                        n2621 = local read "EVENT LOG"() -> (w3165:string)
                        n2622 = call "Event Log.vi"("Content"="Test in progress", "EVENT LOG"=w3165) -> ("EVENT LOG"=w3167:string)  [unwired: 8 in, 1 out]
                        n2623 = local write "EVENT LOG"(w3167) -> ()
                      }
                    }
                    n2624 = disable-structure shown="Enabled" {
                      disable-tunnel: [w3156 w3162] -> w3145
                      frame Disabled {
                        n2625 = local read "Set Hz"() -> (w3159:dbl)
                        n2626 = call <vilib>:"Uniform White Noise Waveform.vi"() -> ("signal out"=w3158:waveform(dbl))  [unwired: 10 in, 1 out]
                        n2627 = Random Number (0-1)() -> (number: 0 to 1=w3155:dbl)
                        n2628 = Add(x=w3159, y=w3158) -> (x+y=w3157:waveform(dbl))
                        n2629 = Multiply(x=ext 0.01 ("y"), y=w3155) -> (x*y=w3153:ext)
                        n2630 = Multiply(x=w3157, y=w3153) -> (x*y=w3156:waveform(ext))
                      }
                      frame Enabled {
                        n2631 = call-poly <vilib>:"Random Number (Range).vi"("lower bound (0)"=49.89, "upper bound (100)"=50.8) -> ("number"=w3162:dbl)  [unwired: 9 in]
                      }
                    }
                    "StartFlg" <- TRUE ("StartFlg")
                  }
                }
                n2632 = case shown="True" w3115 {
                  frame False {
                  }
                  frame True {
                    n2633 = local write "clk"(10.0 ("clk")) -> ()
                    n2634 = Get Date/Time In Seconds() -> (seconds since 1Jan1904=w3170:timestamp)
                    n2635 = To Double Precision Float(number=w3170) -> (double precision float=w3168:dbl)
                    n2636 = local write "acq timer"(w3168) -> ()
                    n2637 = local write "act save time"(w3168) -> ()
                  }
                }
                n2638 = call "Elapsed Time"("Time Target (s)"="Countdown", "Reset"=w3104) -> ("Elapsed Time (s)"=w3109:dbl, "Time has Elapsed"=w3107:bool)  [unwired: 10 in, 6 out]
                "Countdown 2" <- w3109
                n2639 = Subtract(x=w3109, y=2.0) -> (x-y=w3112:dbl)
                n2640 = Less?(x=w3112, y="Countdown") -> (x < y?=w3110:bool)
                n2641 = And(x=w3110, y=w3107) -> (x .and. y?=w3106:bool)
                n2642 = case shown="True" w3106 {
                  frame False {
                  }
                  frame True {
                    (unwired) dbl[] [] ("History Data")
                    n2643 = local write "Engage"(FALSE ("Engage")) -> ()
                    n2644 = local write "RUN"(TRUE ("RUN")) -> ()
                    n2645 = local read "Humidity ( %RH )"() -> (→"Rh Before":dbl)
                  }
                }
                n2646 = local read "Test \nStatus"() -> (w3102:bool)
                n2647 = Select(t=w3100, s=w3102, f=0.0) -> (s? t:f=w3101:dbl)
                n2648 = local write "Frequency ( Hz )"(w3101) -> ()
              }
              frame #1 {
                w3193 = 1000000.0 ("x")
                # "HC;1/0\nST;VALUE"
                # "Elapsed time\ncof\nstroke\nAir temp\nTemp\nHumidity"
                # "acq timer\n\nact save time"
                # "convert to microseconds"
                n2649 = local read "COUNT"() -> (w3176:i32)
                n2650 = local read "Rate"() -> (w3189:dbl)
                n2651 = Divide(x=w3193, y=w3189) -> (x/y=w3194:dbl)
                n2652 = Greater Or Equal?(x=w3176, y=250) -> (x >= y?=w3175:bool)
                n2653 = Get Date/Time In Seconds() -> (seconds since 1Jan1904=w3196:timestamp)
                n2654 = case shown="True" w3175 {
                  frame False {
                    n2655 = local read "COUNT"() -> (w3197:i32)
                    n2656 = Increment(x=w3197) -> (x+1=w3198:i32)
                    n2657 = local write "COUNT"(w3198) -> ()
                  }
                  frame True {
                    n2658 = local write "COUNT"(0 ("COUNT")) -> ()
                  }
                }
                n2659 = local read "Samplingtime 2"() -> (w3174:dbl)
                n2660 = local read "act save time"() -> (w3191:dbl)
                n2661 = Divide(x=w3194, y=w3193) -> (x/y=w3192:dbl)
                n2662 = To Double Precision Float(number=w3196) -> (double precision float=w3185:dbl)
                n2663 = Add(x=w3191, y=w3174) -> (x+y=w3190:dbl)
                n2664 = local read "acq timer"() -> (w3195:dbl)
                n2665 = local read "COUNT"() -> (w3178:i32)
                n2666 = Greater Or Equal?(x=w3185, y=w3190) -> (x >= y?=w3173:bool)
                n2667 = Multiply(x=w3192, y=w3178) -> (x*y=w3184:dbl)
                n2668 = Subtract(x=w3185, y=w3195) -> (x-y=w3187:dbl)
                n2669 = local read "Save"() -> (w3188:bool)
                n2670 = Add(x=w3187, y=w3184) -> (x+y=w3171:dbl)
                "Elapsed time 3" <- w3171
                n2671 = And(x=w3173, y=w3188) -> (x .and. y?=w3186:bool)
                n2672 = Divide(x=w3171, y=60.0) -> (x/y=w3182:dbl)
                n2673 = local read "Test \nStatus"() -> (w3172:bool)
                n2674 = local read "clk"() -> (w3179:dbl)
                n2675 = Equal?(x=w3179, y=10.0) -> (x = y?=w3181:bool)
                n2676 = case shown="True" w3186 {
                  tunnel: w3185 -> [_ w3312]
                  tunnel: [FALSE ("Boolean 2") TRUE ("Boolean 2")] -> _
                  frame False {
                  }
                  frame True {
                    w3266 = ";" ("Substring")
                    # "Pid out/\nFreq response value"
                    n2677 = local write "act save time"(w3312) -> ()
                    n2678 = local read "FILE"() -> (w3260:string)
                    n2679 = call "file check.vi"("file name in"=w3260) -> ("error out"=w3263:errorcluster, "file name out"=w3258:string)  [unwired: 9 in]
                    n2680 = local read "LVDT STROKE"() -> (w3255:dbl)
                    n2681 = local read "Add up Stroke"() -> (w3253:dbl)
                    n2682 = call "FILE PATH CREATION.vi"("error in"=w3263, "FILE NAME :"=w3258) -> ("FILE OUT"=w3261:path)  [unwired: 8 in, 1 out]
                    n2683 = local read "STROKE Initialize"() -> (w3248:bool)
                    n2684 = Concatenate Strings(w3258, ".dgf" ("Substring")) -> (w3262:string)
                    n2685 = Subtract(x=w3255, y=w3253) -> (x-y=w3254:dbl)
                    n2686 = Absolute Value(x=w3254) -> (abs(x)=w3251:dbl)